vi "IMAQdx_AbsImage_Flea3_v4.5.vi"() -> ()   [LabVIEW 2013] (continued)
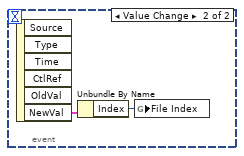
[diagram p3: hidden frame]
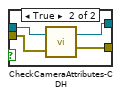
[diagram p5: hidden frame]
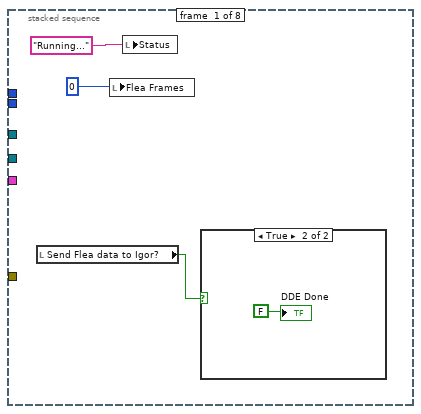
[diagram p6: hidden frame]
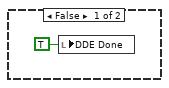
[diagram p7: hidden frame]
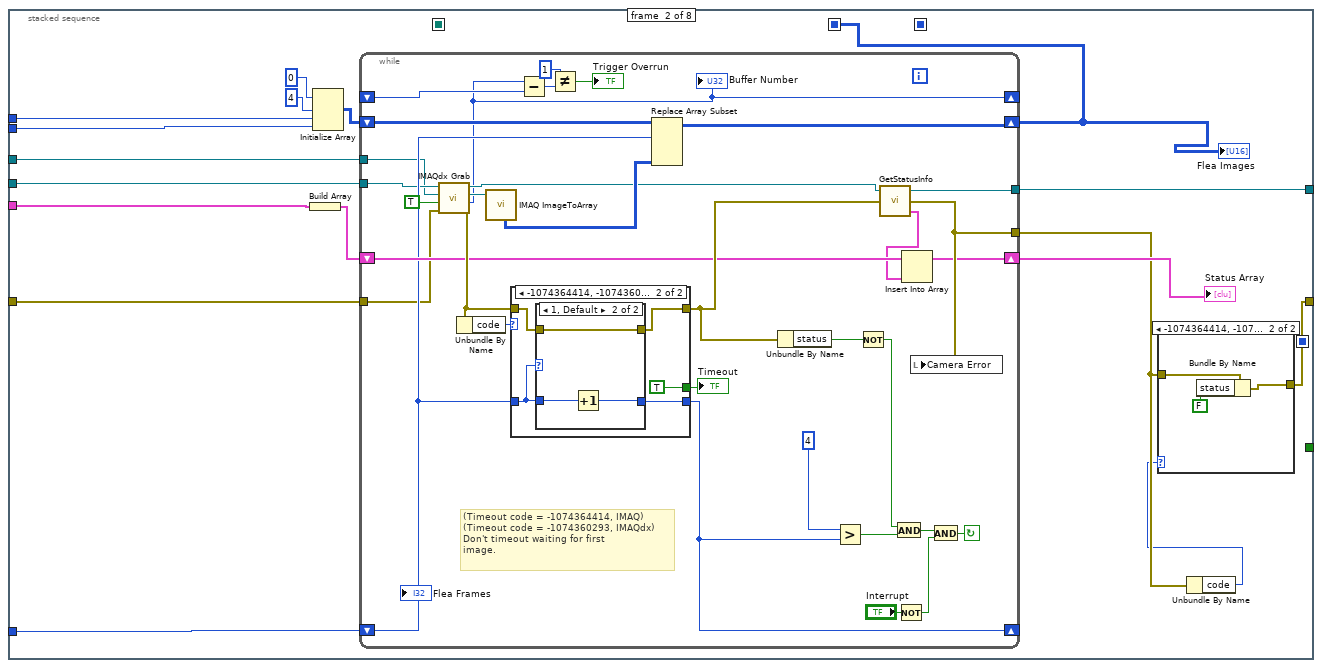
[diagram p8: hidden frame]
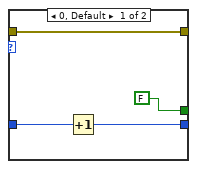
[diagram p10: hidden frame]
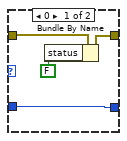
[diagram p11: hidden frame]
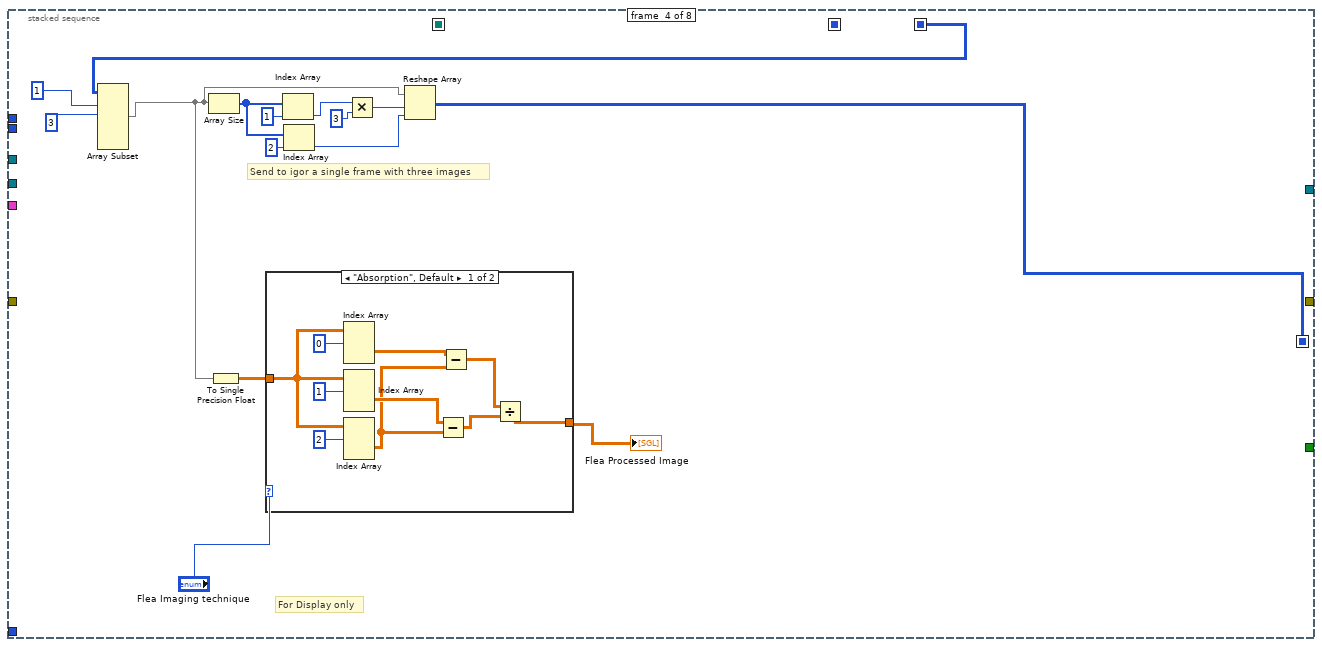
[diagram p14: hidden frame]
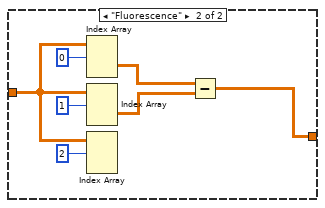
[diagram p15: hidden frame]
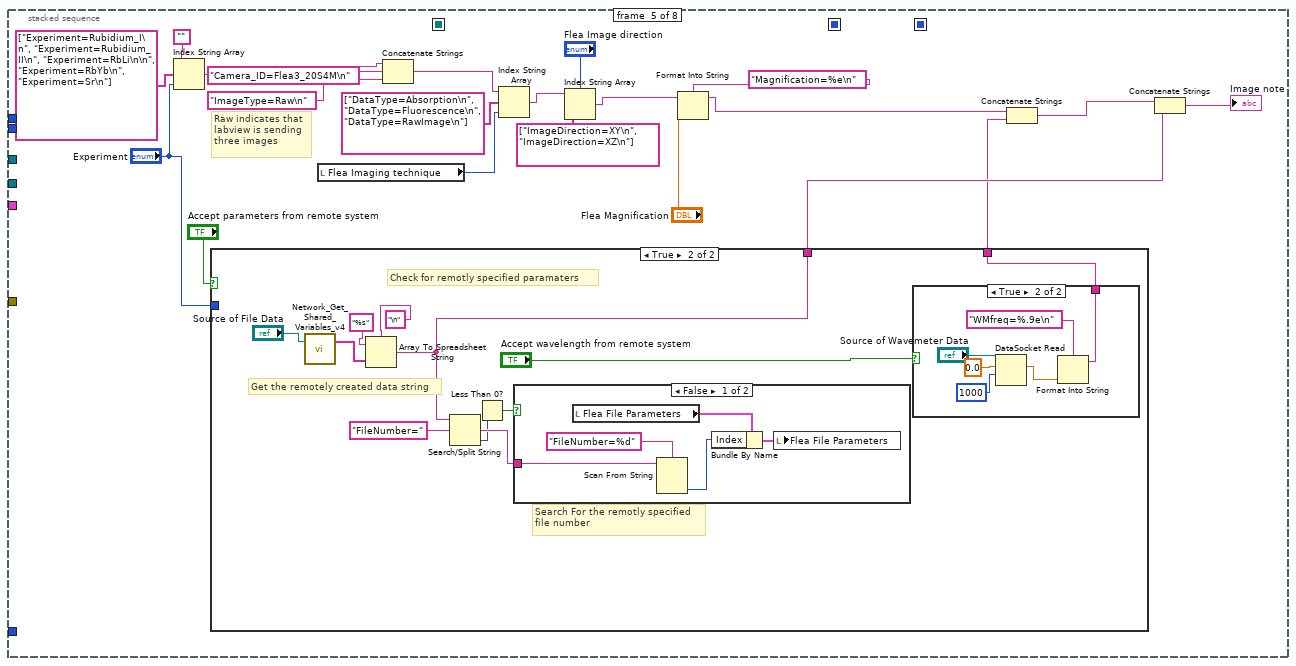
[diagram p16: hidden frame]
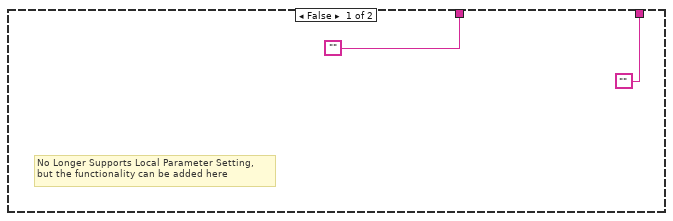
[diagram p17: hidden frame]
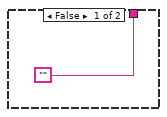
[diagram p18: hidden frame]
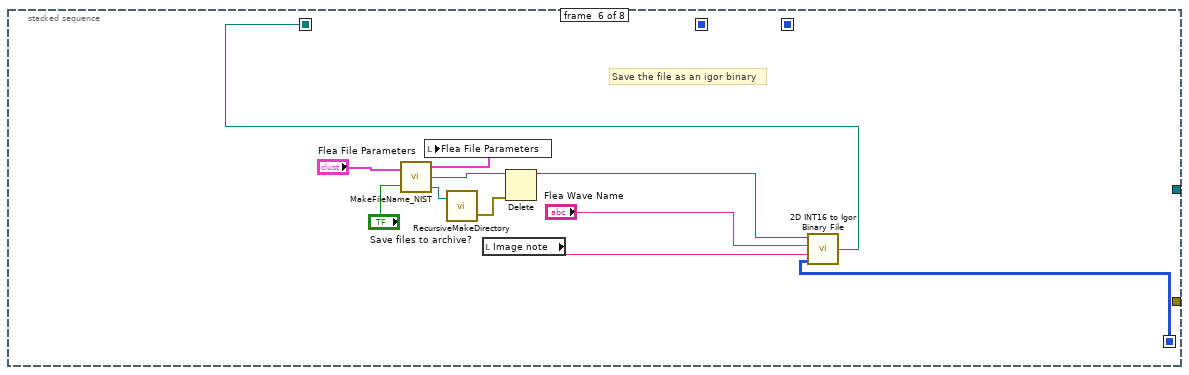
[diagram p20: hidden frame]
                  frame "Absorption", Default {
                    n59 = Index Array(array=w186, index (dim 0)=0 ("Number of buffers")) -> (element=w185:sgl[][])  [unwired: 2 in]
                    n60 = Index Array(array=w186, index (dim 0)=1 ("Number of buffers")) -> (element=w184:sgl[][])  [unwired: 2 in]
                    n61 = Index Array(array=w186, index (dim 0)=2 ("Number of buffers")) -> (element=w183:sgl[][])  [unwired: 2 in]
                    n62 = Subtract(x=w184, y=w183) -> (x-y=w182:sgl[][])
                    n63 = Subtract(x=w185, y=w183) -> (x-y=w181:sgl[][])
                    n64 = Divide(x=w181, y=w182) -> (x/y=w187:sgl[][])
                  }
                  frame "Fluorescence" {
                    n65 = Index Array(array=w194, index (dim 0)=0 ("Number of buffers")) -> (element=w192:sgl[][])  [unwired: 2 in]
                    n66 = Index Array(array=w194, index (dim 0)=1 ("Number of buffers")) -> (element=w191:sgl[][])  [unwired: 2 in]
                    n67 = Index Array(array=w194, index (dim 0)=2 ("Number of buffers")) -> ()  [unwired: 2 in, 1 out]
                    n68 = Subtract(x=w192, y=w191) -> (x-y=w193:sgl[][])
                  }
                }
                "Flea Processed Image" <- w179
                n69 = Index Array(array=w174, index=1 ("Number of buffers")) -> (element=w171:i32)
                n70 = Index Array(array=w174, index=2 ("Number of buffers")) -> (element=w170:i32)
                n71 = Multiply(x=w171, y=3 ("Number of buffers")) -> (x*y=w176:i32)
                n72 = Reshape Array(w166, w176, w170) -> (w178:u16[][])
              }
              frame #4 {
                # "Raw indicates that\nlabview is sending\nthree images"
                n73 = Index String Array(1:"Experiment", 2:string[] ["Experiment=Rubidium_I\n", "Experiment=Rubidium_II\n", "Experiment=RbLi\n\n", "Experiment=RbYb\n", "Experiment=Sr\n"], 3:"") -> (0:w206:string)
                n74 = case shown="True" "Accept parameters from remote system" {
                  tunnel: ["" w224] -> w211
                  tunnel: "Experiment" -> [_ _]
                  tunnel: ["" w221] -> w198
                  frame False {
                    # "No Longer Supports Local Parameter Setting,\nbut the functionality can be added here"
                  }
                  frame True {
                    # "Check for remotly specified paramaters"
                    # "Get the remotely created data string"
                    # "Search For the remotly specified\nfile number"
                    n75 = call "Network_Get_Shared_Variables_v4.vi"("Source of Data"="Source of File Data") -> ("Igor Instruction String"=w231:string[])  [unwired: 1 in, 1 out]
                    n76 = Array To Spreadsheet String(delimiter (Tab)="\n", array=w231, 3:"%s") -> (spreadsheet string=w224:string)
                    n77 = Search/Split String(string=w224, search string/char (-)="FileNumber=") -> (match + rest of string=w227:string, offset of match=w226:i32)  [unwired: 2 out]
                    n78 = Less Than 0?(x=w226) -> (x < 0?=w225:bool)
                    n79 = case shown="False" w225 {
                      tunnel: w227 -> [w243 _]
                      frame False {
                        n80 = local read "Flea File Parameters"() -> (w241:T1)
                        n81 = Scan From String(format string="FileNumber=%d", input string=w243) -> (output 1=w239:i32)  [unwired: 2 in, 4 out]
                        n82 = Bundle By Name(cluster=w241, "Index"=w239) -> (w240:T1)
                        n83 = local write "Flea File Parameters"(w240) -> ()
                      }
                      frame True {
                      }
                    }
                    n84 = case shown="True" "Accept wavelength from remote system" {
                      tunnel: ["" w233] -> w221
                      frame False {
                      }
                      frame True {
                        n85 = DataSocket Read(9:1000 ("ms timeout (10000)"), 10:0.0, 11:"Source of Wavemeter Data") -> (2:w236:dbl)  [unwired: 2 in, 6 out]
                        n86 = Format Into String(format string="WMfreq=%.9e\n", w236) -> (resulting string=w233:string)  [unwired: 2 in, 1 out]
                      }
                    }
                  }
                }
                n87 = local read "Flea Imaging technique"() -> (w215:enum16{"Absorption", "Fluorescence", "RawImage"})
                n88 = Concatenate Strings(w206, "Camera_ID=Flea3_20S4M\n", "ImageType=Raw\n") -> (w207:string)
                n89 = Index String Array(1:w215, 2:string[] ["DataType=Absorption\n", "DataType=Fluorescence\n", "DataType=RawImage\n"], 3:w207) -> (0:w216:string)
                n90 = Index String Array(1:"Flea Image direction", 2:string[] ["ImageDirection=XY\n", "ImageDirection=XZ\n"], 3:w216) -> (0:w218:string)
                n91 = Format Into String(format string="Magnification=%e\n", initial string=w218, "Flea Magnification") -> (resulting string=w199:string)  [unwired: 1 in, 1 out]
                n92 = Concatenate Strings(w199, w198) -> (w200:string)
                n93 = Concatenate Strings(w200, w211) -> (→"Image note":string)
              }
              frame #5 {
                # "Save the file as an igor binary"
                n94 = call "MakeFileName_NIST.vi"("File Parameters"="Flea File Parameters", "Save permanent file?"="Save files to archive?") -> ("New file parameters."=w250:T1, "Path to File"=w252:path, "path"=w251:path)
                n95 = local write "Flea File Parameters"(w250) -> ()
                n96 = call "RecursiveMakeDirectory.vi"("Directory to create"=w251) -> ("error out"=w254:errorcluster)  [unwired: 1 in, 1 out]
                n97 = local read "Image note"() -> (w247:string)
                n98 = Delete(path (use dialog)=w252, error in=w254) -> (deleted path=w245:path)  [unwired: 5 out]
                n99 = call "2D INT16 to Igor Binary File.vi"("Wave Data (I16)"=w248, "Wave Note (\"\")"=w247, "WaveName"="Flea Wave Name", "Path (default: dialog)"=w245) -> ("Path chosen"=w244:path)
              }
              frame #6 {
                # "Be sure the file is written"
                n100 = Wait (ms)(milliseconds to wait=u32 10) -> ()  [unwired: 1 out]
              }
              frame #7 {
                n101 = case shown="True" "Send Flea data to Igor?" {
                  tunnel: w258 -> [_ w270]
                  tunnel: ["" w262] -> w257
                  frame False {
                  }
                  frame True {
                    n102 = local read "Send PIXIS data to Igor?"() -> (w265:bool)
                    n103 = flat-sequence {
                      tunnel: w261 -> [w271]
                      frame #0 {
                        # "Tell Igor what file to open"
                        n104 = call <vilib>:"DDE Open Conversation.vi"("topic"="Igor", "service"="Igor") -> ("error out"=w275:errorcluster, "conversation refnum"=w277:u32)  [unwired: 1 in, 5 out]
                        n105 = call <vilib>:"DDE Execute.vi"("error in (no error)"=w275, "command"=w271, "conversation refnum in"=w277) -> ("error out"=w276:errorcluster, "conversation refnum out"=w278:u32)  [unwired: 5 out]
                        n106 = call <vilib>:"DDE Close Conversation.vi"("error in (no error)"=w276, "conversation refnum"=w278) -> ("error out"=→"DDE Error":errorcluster)  [unwired: 7 out]
                      }
                      frame #1 {
                        n107 = local write "DDE Done"(TRUE ("Waiting for Flea File")) -> ()
                      }
                      frame #2 {
                        n108 = Wait (ms)(milliseconds to wait=u32 10) -> ()  [unwired: 1 out]
                      }
                    }
                    n109 = Path To String(path=w270) -> (string=w269:string)
                    n110 = Search and Replace String(replace all?=TRUE, input string=w269, search string="\\", replace string="\\\\") -> (result string=w264:string)  [unwired: 1 in, 6 out]
                    n111 = case shown="True" w265 {
                      tunnel: w264 -> [w283 w287]
                      tunnel: "Flea Data Series Name" -> [w284 w290]
                      tunnel: [w281 w288] -> w262
                      tunnel: [w281 w288] -> w261
                      frame False {
                        n112 = Format Into String(format string="AutoRunV3(\"%s\",\"%s\") ", w284, w283) -> (resulting string=w281:string)  [unwired: 2 in, 1 out]
                      }
                      frame True {
                        n113 = local read "PIXIS Data Series Name"() -> (w286:string)
                        n114 = stacked-sequence {
                          tunnel: [_ w293] -> w285
                          frame #0 {
                            n115 = while {
                              stop <- w292 continue-if-true
                              n116 = local read "Waiting for PIXIS file"() -> (w292:bool)
                              n117 = Wait (ms)(milliseconds to wait=u32 5) -> ()  [unwired: 1 out]
                            }
                          }
                          frame #1 {
                            n118 = local read "PIXIS Path"() -> (w298:path)
                            n119 = Path To String(path=w298) -> (string=w294:string)
                            n120 = Search and Replace String(replace all?=TRUE, input string=w294, search string="\\", replace string="\\\\") -> (result string=w293:string)  [unwired: 1 in, 6 out]
                          }
                        }
                        n121 = Format Into String(format string="AutoRunV4(\"%s\",\"%s\",\"%s\",\"%s\") ", w290, w287, w286, w285) -> (resulting string=w288:string)  [unwired: 2 in, 1 out]
                      }
                    }
                  }
                }
                "Command to Igor" <- w257
                "Flea Path" <- w258
              }
            }
            "Flea Loop" <- w75
          }
          n122 = call <vilib>:"IMAQdx Unconfigure Acquisition.vi"("error in"=w34, "Session In"=w31) -> ("error out"=w33:errorcluster, "Session Out"=w30:T2)  [unwired: 8 in]
          n123 = call <vilib>:"IMAQdx Close Camera.vi"("error in"=w33, "Session In"=w30) -> ("error out"=w32:errorcluster)  [unwired: 9 out]
        }
      }
      n124 = case shown="True" w23 {
        tunnel: w25 -> [w299 w301]
        tunnel: [w299 w300] -> w24
        frame False {
        }
        frame True {
          n125 = while {
            tunnel: [w303] -> w300
            tunnel: w301 -> [w305]
            i -> [w306]
            stop <- w304 stop-if-true
            n126 = stacked-sequence {
              seq-local: [_ _ w355 _ _ _ _] -> [_ _ _ _ w413 _ _]
              seq-local: [_ _ _ _ w409 _ _] -> [_ _ _ _ _ _ w429]
              seq-local: [_ w313 _ _ _ _ _] -> [_ _ w343 _ _ _ _]
              seq-local: [_ w311 _ _ _ _ _] -> [_ _ _ _ _ _ w423]
              seq-local: [_ w310 _ _ _ _ _] -> [_ _ _ _ _ _ w422]
              tunnel: w305 -> [_ w312 _ _ _ _ _]
              tunnel: [_ _ _ _ _ _ w424] -> w304
              tunnel: [_ _ _ _ _ _ w421] -> w303
              tunnel: [_ _ _ _ _ _ w420] -> w302
              frame #0 {
                n127 = local write "Status"("Running...") -> ()
                n128 = local write "PIXIS Frames"(i64 0) -> ()
                "Waiting for PIXIS file" <- TRUE
              }
              frame #1 {
                n129 = while {
                  tunnel: "SPE File Path" -> [w333]
                  shift-right: [w332] -> w323
                  shift-left: w312 -> [w329]
                  tunnel: [w330] -> w315
                  tunnel: "Source of Control Data" -> [w325]
                  stop <- w331 stop-if-true
                  n130 = local read "CycleDone"() -> (w328:bool)
                  n131 = DataSocket Read(8:w329, 10:w328, 11:w325) -> (0:w327:errorcluster, 2:w326:bool)  [unwired: 2 in, 5 out]
                  "CycleDone" <- w326
                  "DS Error" <- w327
                  n132 = case shown="True" w326 {
                    tunnel: w333 -> [w336 w341]
                    tunnel: [w335 w340] -> w332
                    tunnel: [FALSE ("file or folder exists?") w339] -> w331
                    tunnel: [w336 w338] -> w330
                    tunnel: w327 -> [w335 w337]
                    frame False {
                    }
                    frame True {
                      n133 = call <vilib>:"Check if File or Folder Exists.vi"("error in (no error)"=w337, "path"=w341) -> ("error out"=w340:errorcluster, "file or folder exists?"=w339:bool, "dup path"=w338:path)  [unwired: 7 in]
                    }
                  }
                }
                n134 = call "Load SPE v0.2.vi"("Error In"=w323, "File Path In"=w315) -> ("Error Out"=w310:errorcluster, "DataBlock Info"=w317:T5, "Output Stack"=w320:cluster{u16[][][]}[], "File Path Out"=w311:path, "Parse Errors"=→"XML Parse Errors":string)  [unwired: 5 in]
                "DataBlock Info" <- w317
                n135 = Unbundle By Name(w317) -> ("frame count"=→"PIXIS Frames":i64)
                n136 = Index Array(array=w320, index=0) -> (element=w318:cluster{u16[][][]})
                n137 = Array Size(array=w320) -> (size(s)=→"Data Array Size":i32)
                n138 = Unbundle(w318) -> (w313:u16[][][])
                "PIXIS Images" <- w313
              }
              frame #2 {
                # "Send to igor a single frame with three images"
                # "For Display only"
                n139 = Array Subset(array=w343, index (dim 0)=1 ("index"), length (dim 0)=3 ("length")) -> (w344:u16[][][])  [unwired: 4 in]
                n140 = Array Size(array=w344) -> (size(s)=w351:i32[])
                n141 = To Single Precision Float(number=w344) -> (single precision float=w352:sgl[][][])
                n142 = case shown="\"Absorption\", Default" "PIXIS Imaging technique" {
                  tunnel: [w362 w369] -> w342
                  tunnel: w352 -> [w363 w370]
                  frame "Absorption", Default {
                    n143 = Index Array(array=w363, index (dim 0)=0 ("Number of buffers")) -> (element=w359:sgl[][])  [unwired: 2 in]
                    n144 = Index Array(array=w363, index (dim 0)=1 ("Number of buffers")) -> (element=w357:sgl[][])  [unwired: 2 in]
                    n145 = Index Array(array=w363, index (dim 0)=2 ("Number of buffers")) -> (element=w358:sgl[][])  [unwired: 2 in]
                    n146 = Subtract(x=w357, y=w358) -> (x-y=w361:sgl[][])
                    n147 = Subtract(x=w359, y=w358) -> (x-y=w360:sgl[][])
                    n148 = Divide(x=w360, y=w361) -> (x/y=w362:sgl[][])
                  }
                  frame "Fluorescence" {
                    n149 = Index Array(array=w370, index (dim 0)=0 ("Number of buffers")) -> (element=w368:sgl[][])  [unwired: 2 in]
                    n150 = Index Array(array=w370, index (dim 0)=1 ("Number of buffers")) -> (element=w367:sgl[][])  [unwired: 2 in]
                    n151 = Index Array(array=w370, index (dim 0)=2 ("Number of buffers")) -> ()  [unwired: 2 in, 1 out]
                    n152 = Subtract(x=w368, y=w367) -> (x-y=w369:sgl[][])
                  }
                }
                "PIXIS Processed Image" <- w342
                n153 = Index Array(array=w351, index=1 ("Number of buffers")) -> (element=w348:i32)
                n154 = Index Array(array=w351, index=2 ("Number of buffers")) -> (element=w347:i32)
                n155 = Multiply(x=w348, y=3 ("Number of buffers")) -> (x*y=w353:i32)
                n156 = Reshape Array(w344, w353, w347) -> (w355:u16[][])
              }
              frame #3 {
                # "Raw indicates that\nlabview is sending\nthree images"
                n157 = local read "Accept parameters from remote system"() -> (w374:bool)
                n158 = local read "Experiment"() -> (w375:T3)
                n159 = Index String Array(1:w375, 2:string[] ["Experiment=Rubidium_I\n", "Experiment=Rubidium_II\n", "Experiment=RbLi\n\n", "Experiment=RbYb\n", "Experiment=Sr\n"], 3:"") -> (0:w379:string)
                n160 = case shown="True" w374 {
                  tunnel: ["" w395] -> w384
                  tunnel: w375 -> [_ _]
                  frame False {
                    # "No Longer Supports Local Parameter Setting,\nbut the functionality can be added here"
                  }
                  frame True {
                    # "Check for remotely specified paramaters"
                    # "Get the remotely created data string"
                    # "Search For the remotly specified\nfile number"
                    n161 = local read "Source of File Data"() -> (w394:refnum<k21>)
                    n162 = call "Network_Get_Shared_Variables_v4.vi"("Source of Data"=w394) -> ("Igor Instruction String"=w402:string[])  [unwired: 1 in, 1 out]
                    n163 = Array To Spreadsheet String(delimiter (Tab)="\n", array=w402, 3:"%s") -> (spreadsheet string=w395:string)
                    n164 = Search/Split String(string=w395, search string/char (-)="FileNumber=") -> (match + rest of string=w398:string, offset of match=w397:i32)  [unwired: 2 out]
                    n165 = Less Than 0?(x=w397) -> (x < 0?=w396:bool)
                    n166 = case shown="False" w396 {
                      tunnel: w398 -> [w407 _]
                      frame False {
                        n167 = Scan From String(format string="FileNumber=%d", input string=w407) -> (output 1=w403:i32)  [unwired: 2 in, 4 out]
                        n168 = local read "PIXIS File Parameters"() -> (w405:T1)
                        n169 = Bundle By Name(cluster=w405, "Index"=w403) -> (w404:T1)
                        n170 = local write "PIXIS File Parameters"(w404) -> ()
                      }
                      frame True {
                      }
                    }
                  }
                }
                n171 = local read "PIXIS Imaging technique"() -> (w389:enum16{"Absorption", "Fluorescence", "RawImage"})
                n172 = Concatenate Strings(w379, "Camera_ID=PIXIS\n", "ImageType=Raw\n") -> (w380:string)
                n173 = Index String Array(1:w389, 2:string[] ["DataType=Absorption\n", "DataType=Fluorescence\n", "DataType=RawImage\n"], 3:w380) -> (0:w390:string)
                n174 = Index String Array(1:"PIXIS Image direction", 2:string[] ["ImageDirection=XY\n", "ImageDirection=XZ\n"], 3:w390) -> (0:w392:string)
                n175 = Format Into String(format string="Magnification=%e\n", initial string=w392, "PIXIS Magnification") -> (resulting string=w386:string)  [unwired: 1 in, 1 out]
                n176 = Concatenate Strings(w386, w384) -> (→"PIXIS Image Note":string)
              }
              frame #4 {
                # "Save the file as an igor binary"
                n177 = local read "Save files to archive?"() -> (w408:bool)
                n178 = call "MakeFileName_NIST.vi"("File Parameters"="PIXIS File Parameters", "Save permanent file?"=w408) -> ("New file parameters."=w415:T1, "Path to File"=w417:path, "path"=w416:path)
                n179 = local write "PIXIS File Parameters"(w415) -> ()
                n180 = call "RecursiveMakeDirectory.vi"("Directory to create"=w416) -> ("error out"=w418:errorcluster)  [unwired: 1 in, 1 out]
                n181 = local read "PIXIS Image Note"() -> (w412:string)
                n182 = Delete(path (use dialog)=w417, error in=w418) -> (deleted path=w410:path)  [unwired: 5 out]
                n183 = call "2D INT16 to Igor Binary File.vi"("Wave Data (I16)"=w413, "Wave Note (\"\")"=w412, "WaveName"="PIXIS Wave Name", "Path (default: dialog)"=w410) -> ("Path chosen"=w409:path)
              }
              frame #5 {
                # "Be sure the file is written"
                n184 = Wait (ms)(milliseconds to wait=u32 10) -> ()  [unwired: 1 out]
              }
              frame #6 {
                n185 = local read "Send Flea data to Igor?"() -> (w425:bool)
                n186 = Not(x=w425) -> (.not. x?=w428:bool)
                n187 = And(x="Send PIXIS data to Igor?", y=w428) -> (x .and. y?=w426:bool)
                n188 = case shown="False" w426 {
                  tunnel: w429 -> [_ w453]
                  tunnel: w423 -> [w432 w442]
                  tunnel: w422 -> [w431 w443]
                  tunnel: [w433 w444] -> w421
                  tunnel: [w430 w441] -> w420
                  frame False {
                    n189 = stacked-sequence {
                      tunnel: [w437 _] -> w433
                      tunnel: w432 -> [w436 _]
                      tunnel: w431 -> [w435 _]
                      tunnel: [w434 _] -> w430
                      frame #0 {
                        n190 = local write "Waiting for PIXIS file"(FALSE ("Waiting for PIXIS file")) -> ()
                        n191 = Delete(path (use dialog)=w436, error in=w435) -> (deleted path=w434:path, error out=w437:errorcluster)  [unwired: 3 in, 1 out]
                      }
                      frame #1 {
                        n192 = while {
                          stop <- w439 stop-if-true
                          n193 = local read "DDE Done"() -> (w439:bool)
                          n194 = Wait (ms)(milliseconds to wait=u32 5) -> ()  [unwired: 1 out]
                        }
                      }
                    }
                  }
                  frame True {
                    # "Tell Igor what file to open"
                    n195 = Path To String(path=w453) -> (string=w452:string)
                    n196 = call <vilib>:"DDE Open Conversation.vi"("topic"="Igor", "service"="Igor") -> ("error out"=w457:errorcluster, "conversation refnum"=w455:u32)  [unwired: 1 in, 5 out]
                    n197 = Search and Replace String(replace all?=TRUE, input string=w452, search string="\\", replace string="\\\\") -> (result string=w448:string)  [unwired: 1 in, 6 out]
                    n198 = Format Into String(format string="AutoRunV3(\"%s\",\"%s\") ", "PIXIS Data Series Name", w448) -> (resulting string=w446:string)  [unwired: 2 in, 1 out]
                    n199 = call <vilib>:"DDE Execute.vi"("error in (no error)"=w457, "command"=w446, "conversation refnum in"=w455) -> ("error out"=w456:errorcluster, "conversation refnum out"=w454:u32)  [unwired: 5 out]
                    n200 = local write "Command to Igor"(w446) -> ()
                    n201 = call <vilib>:"DDE Close Conversation.vi"("error in (no error)"=w456, "conversation refnum"=w454) -> ("error out"=w445:errorcluster)  [unwired: 7 out]
                    n202 = local write "DDE Error"(w445) -> ()
                    n203 = Delete(path (use dialog)=w442, error in=w443) -> (deleted path=w441:path, error out=w444:errorcluster)  [unwired: 3 in, 1 out]
                  }
                }
                n204 = local read "stop"() -> (w424:bool)
                "PIXIS Path" <- w429
              }
            }
            "SPE delete path" <- w302
            "PIXIS Loop" <- w306
          }
        }
      }
    }
    frame #2 {
      n205 = local write "stop"(FALSE ("stop")) -> ()
      n206 = local write "Status"("Done.") -> ()
      "Camera Error" <- w462
      "SPE Load Error Out" <- w463
    }
    frame #3 {
      n207 = Stop() -> ()  [unwired: 1 out]
    }
  }
  n208 = while {
    stop <- TRUE continue-if-true
    n209 = event shown="[0] \"Flea Raw image to view\", \"Flea Images\", \"Update Graphics\", \"PIXIS Raw image to view\", \"PIXIS Images\": Value Change;  Timeout" {
      selector: _ -> [_ _]
      dyn-events: _ -> [_ _]
      timeout: 1000 -> [_ _]
      event "Flea Raw image to view", "Flea Images", "Update Graphics", "PIXIS Raw image to view", "PIXIS Images": Value Change; Timeout {
        n210 = event-data() -> ()  [unwired: 4 out]
        n211 = case shown="True" "Update Graphics" {
          frame False {
          }
          frame True {
            n212 = local read "Flea Images"() -> (w473:u16[][][])
            n213 = local read "PIXIS Images"() -> (w468:u16[][][])
            n214 = Index Array(array=w473, index (dim 0)="Flea Raw image to view") -> (element=→"Flea Raw Image":u16[][])  [unwired: 2 in]
            n215 = Index Array(array=w468, index (dim 0)="PIXIS Raw image to view") -> (element=→"PIXIS Raw Image":u16[][])  [unwired: 2 in]
          }
        }
      }
      event Value Change {
        n216 = event-data() -> ("NewVal"=w474:T1)  [unwired: 6 out]
        n217 = Unbundle By Name(w474) -> ("Index"=w475:u32)
        n218 = global write "FileInfo_Global.vi" "File Index"(w475) -> ()
      }
    }
  }
